vi "UHR-Fleezers Control (host) - 10.4.vi"() -> ()   [LabVIEW 2010] (continued)
              }
              frame #4 {
                n1609 = call "Write to pump.vi"("string"="start", "VISA resource name"=w7308) -> ()  [unwired: 1 out]
              }
            }
          }
        }
      }
      event "Inject Pump 2": Value Change {
        n1610 = event-data() -> ()  [unwired: 7 out]
        n1611 = local read "Pump write delay (ms)"() -> (w7312:dbl)
        n1612 = flat-sequence {
          tunnel: w7310 -> [w7325]
          tunnel: w7312 -> [w7321]
          tunnel: "Inject Pump 2" -> [_]
          tunnel: w7312 -> [w7327]
          tunnel: w7310 -> [w7328]
          frame #0 {
            n1613 = local read "All Pump Parameters"() -> (w7320:T6)
            n1614 = Multiply(x=60.0, y="Flush Center Ch Rate (ul/m)") -> (x*y=w7317:dbl)
            n1615 = Unbundle By Name(w7320) -> ("Pump 2"=w7326:T49)
            n1616 = call "Set pump parameters.vi"("Pump write delay (ms)"=w7321, "Volume (uL)"="Flush Center Ch Volume (uL)", "Rate (uL/h)"=w7317, "Units"=3.0, "Pump #"=2.0, "Pump Parameters In"=w7326, "VISA resource name"=w7325) -> ("Pump Parameters Out"=w7319:T49)  [unwired: 3 in]
            n1617 = Bundle By Name(cluster=w7320, "Pump 2"=w7319) -> (w7318:T6)
            n1618 = local write "All Pump Parameters"(w7318) -> ()
            n1619 = Add(x="Flush Center Ch Volume (uL)", y="Total Volume\nFlushed (uL)") -> (x+y=w7314:dbl)
            n1620 = local write "Total Volume\nFlushed (uL)"(w7314) -> ()
          }
          frame #1 {
            n1621 = Wait (ms)(milliseconds to wait=w7327) -> ()  [unwired: 1 out]
          }
          frame #2 {
            n1622 = call "Write to pump.vi"("string"="start", "VISA resource name"=w7328) -> ()  [unwired: 1 out]
          }
        }
        n1623 = local read "Chemyx Syringe Pump Serial Port"() -> (w7310:refnum<visa-resource-name>)
      }
      event "Sample Channel Flow": Value Change {
        n1624 = event-data() -> ()  [unwired: 7 out]
        n1625 = Select(t="run" ("string"), s="Sample Channel Flow", f="stop" ("string")) -> (s? t:f=w7330:string)
        n1626 = Concatenate Strings(w7330, "\r") -> (w7334:string)
        n1627 = VISA Write(VISA resource name=w7336, write buffer=w7334) -> ()  [unwired: 1 in, 3 out]
      }
      event "Flip Green Filter": Value Change {
        n1628 = event-data() -> ()  [unwired: 7 out]
        n1629 = Not(x="Flip Green Filter") -> (.not. x?=w7337:bool)
        n1630 = local write "Flip Green Filter"(w7337) -> ()
        n1631 = flat-sequence {
          tunnel: w7345 -> [w7350]
          tunnel: w7344 -> [w7349]
          tunnel: [w7347] -> w7342
          tunnel: [w7346] -> w7341
          tunnel: [w7390] -> w7340
          tunnel: w7342 -> [w7390]
          tunnel: [w7389] -> w7339
          tunnel: w7341 -> [w7389]
          tunnel: w7340 -> [w7394]
          tunnel: w7339 -> [w7393]
          tunnel: [w7392] -> w7343
          frame #0 {
            n1632 = xnode "Read/Write Control"("FPGA VI Reference In"=w7350, "error in"=w7349, "Green Filter Flipper"=TRUE) -> ("FPGA VI Reference Out"=w7347:T20, "error out"=w7346:errorcluster)
          }
          frame #1 {
            n1633 = Wait (ms)(milliseconds to wait=u32 100) -> ()  [unwired: 1 out]
          }
          frame #2 {
            n1634 = xnode "Read/Write Control"("FPGA VI Reference In"=w7394, "error in"=w7393, "Green Filter Flipper"=FALSE) -> ("error out"=w7392:errorcluster)  [unwired: 1 out]
          }
        }
      }
      event "Pump 1 contents", "Pump 3 contents": Value Change {
        n1635 = event-data() -> ()  [unwired: 7 out]
        n1636 = local read "Pump 1 contents"() -> (→"Pump 1 cont disp":string)
        n1637 = local read "Pump 3 contents"() -> (→"Pump 3 cont disp":string)
      }
      event "Reset Trap Pos. FB": Value Change {
        n1638 = event-data() -> ()  [unwired: 7 out]
        n1639 = xnode "Read/Write Control"("FPGA VI Reference In"=w7438, "error in"=w7437, "Trap Pos. FB Reset"="Reset Trap Pos. FB") -> ()  [unwired: 2 out]
      }
      event "Trap Pos. FB ON": Value Change {
        n1640 = event-data() -> ()  [unwired: 7 out]
        n1641 = xnode "Read/Write Control"("FPGA VI Reference In"=w7479, "error in"=w7478, "Force feedback"="Trap Pos. FB ON") -> ()  [unwired: 2 out]
      }
      event "Trap Pos. FB Range", "Trap Pos. FB Gains", "Trap Pos. FB Mult Factor", "Trap Pos. FB Offset Factor", "Trap Pos FB Negate Action", "Trap Pos FB Monitor\nT1 or T2": Value Change {
        n1642 = event-data() -> ()  [unwired: 7 out]
        n1643 = xnode "Read/Write Control"("FPGA VI Reference In"=w7526, "error in"=w7525, "Trap Pos. FB Range"="Trap Pos. FB Range", "Trap Pos. FB Gains"="Trap Pos. FB Gains", "Trap Pos. FB Mult Factor"="Trap Pos. FB Mult Factor", "Trap Pos. FB Offset Factor"="Trap Pos. FB Offset Factor", "Trap Pos FB Negate Action"="Trap Pos FB Negate Action", "Trap Pos FB Monitor T1 or T2"="Trap Pos FB Monitor\nT1 or T2", "AI1 X Scale"="Trap Pos. AI1 X Pre-scale") -> ()  [unwired: 2 out]
      }
      event "Trap Pos FB SP": Value Change {
        n1644 = event-data() -> ()  [unwired: 7 out]
        n1645 = xnode "Read/Write Control"("FPGA VI Reference In"=w7714, "error in"=w7713, "Trap Pos. FB SP"="Trap Pos FB SP") -> ()  [unwired: 2 out]
      }
      event "Set SP to Reading": Value Change {
        n1646 = event-data() -> ()  [unwired: 7 out]
        n1647 = local read "Trap Pos FB Monitor\nT1 or T2"() -> (w7767:bool)
        n1648 = local read "Trap X AI1 (DMA)"() -> (w7770:T14)
        n1649 = local read "Trap X (AI1)"() -> (w7773:T11)
        n1650 = Unbundle By Name(w7773) -> ("Trap 1"=w7772:fxp<+/-,16,1>, "Trap 2"=w7771:fxp<+/-,16,1>)
        n1651 = Unbundle By Name(w7770) -> ("Set 1"=w7769:fxp<+/-,16,1>, "Set 2"=w7768:fxp<+/-,16,1>)
        n1652 = Select(t=w7772, s=w7767, f=w7771) -> (s? t:f=w7766:fxp<+/-,16,1>)
        n1653 = Select(t=w7769, s=w7767, f=w7768) -> (s? t:f=w7765:fxp<+/-,16,1>)
        n1654 = Not(x="Set SP Using...") -> (.not. x?=w7760:bool)
        n1655 = Select(t=w7766, s=w7760, f=w7765) -> (s? t:f=w7761:fxp<+/-,16,1>)
        n1656 = xnode "Read/Write Control"("FPGA VI Reference In"=w7763, "error in"=w7762, "Trap Pos. FB SP"=w7761) -> ()  [unwired: 2 out]
        n1657 = local write "Trap Pos FB SP"(w7761) -> ()
      }
      event "Trap Pos. FB Out Scale 2^n": Value Change {
        n1658 = event-data() -> ()  [unwired: 7 out]
        n1659 = Scale By Power Of 2(n="Trap Pos. FB Out Scale 2^n", x=ext 1.0) -> (x*2^n=w7820:ext)
        n1660 = property on="Trap Pos. FB Mult Factor" class="DigNum (strict)"("Val(Sgnl)"=w7820) -> ()  [unwired: 2 in, 2 out]
      }
      event "Trap Pos FB Int Count": Value Change {
        n1661 = event-data() -> ()  [unwired: 7 out]
        n1662 = xnode "Read/Write Control"("FPGA VI Reference In"=w7825, "error in"=w7824, "Trap Pos FB Int Count"="Trap Pos FB Int Count") -> ()  [unwired: 2 out]
      }
    }
    "error out 2" <- w4314
    n1663 = node-c288() -> ()  [unwired: 2 out]
  }
  n1664 = timed-loop "Run Scripts, including: stage motion" {
    timing: w57 -> [_]
    timing-out: [_] -> w56
    tunnel: w42 -> [w7864]
    tunnel: w43 -> [w7863]
    stop <- w7865 stop-if-true
    n1665 = node-c288() -> ()  [unwired: 1 in, 1 out]
    n1666 = event shown="[6] \"Dump Beads\": Value Change" {
      selector: _ -> [_ _ _ _ _ _ _ _ _ _ _ _ _ _ _ _]
      dyn-events: _ -> [_ _ _ _ _ _ _ _ _ _ _ _ _ _ _ _]
      timeout: _ -> [_ _ _ _ _ _ _ _ _ _ _ _ _ _ _ _]
      tunnel: ["Set Position" "Move to Position" "Move Cap. 1 (DNA Right)" "Move Cap. 2 (ADig Left)" _ "Cal/Data Acq. Spot" "Dump Beads" "Dip for Protein" _ _ "Got ADig bead" "Got DNA bead" "Take Stepping Data" _ "Take Detection Laser\nImage" _] -> _
      tunnel: [_ _ _ _ _ _ _ _ _ _ _ _ _ _ _ w8280] -> w7865
      tunnel: w7864 -> [_ _ w7906 w7956 _ _ _ _ _ _ _ _ _ _ _ _]
      tunnel: w7863 -> [_ _ w7905 w7957 _ _ _ _ _ _ _ _ _ _ _ _]
      event "Set Position", "Set Position 2", "Set Position 3", "Set Position 4", "Set Position 5", "Set Position 1": Value Change {
        n1667 = event-data() -> ()  [unwired: 1 in, 5 out]
        n1668 = Build Array("Set Position 1", "Set Position 2", "Set Position 3", "Set Position 4", "Set Position 5") -> (w7884:bool[])
        n1669 = Boolean Array To Number(Boolean array=w7884) -> (number=w7883:u32)
        n1670 = Logarithm Base 2(1:w7883) -> (0:w7875:dbl)
        n1671 = call "CONEX_FUNCTIONAL_GLOBAL.vi"("Command"=T23."GET POS") -> ("Current Position"=w7868:dbl[])  [unwired: 8 in, 2 out]
        n1672 = Decrement(x="Position") -> (x-1=w7873:dbl)
        n1673 = Greater Or Equal?(x=w7875, y=0.0) -> (x >= y?=w7876:bool)
        n1674 = Select(t=w7875, s=w7876, f=w7873) -> (s? t:f=w7872:dbl)
        n1675 = Increment(x=w7872) -> (x+1=w7871:dbl)
        n1676 = Build Array (concatenate)(w7871, w7868) -> (w7870:dbl[])
        n1677 = Replace Array Subset(array="Saved Stage Positions", new element=w7870, index (row)=w7872) -> (w7885:dbl[][])  [unwired: 1 in]
        n1678 = local write "Saved Stage Positions"(w7885) -> ()
      }
      event "Move to Position": Value Change {
        n1679 = event-data() -> ()  [unwired: 1 in, 5 out]
        n1680 = flat-sequence {
          frame #0 {
            n1681 = local read "Position"() -> (w7900:dbl)
            n1682 = local read "Saved Stage Positions"() -> (w7898:dbl[][])
            n1683 = Decrement(x=w7900) -> (x-1=w7897:dbl)
            n1684 = Array Subset(array=w7898, index (row)=w7897, length (row)=1 ("length"), index (col)=1 ("index"), length (col)=3 ("length")) -> (w7894:dbl[][])
            n1685 = Reshape Array(w7894, 3 ("dimension size")) -> (w7890:dbl[])
            n1686 = local write "Stage Moving"(TRUE ("Stage Moving")) -> ()
            n1687 = call "CONEX_FUNCTIONAL_GLOBAL.vi"("Axis"=enum16{"X", "Y", "Z", "XY", "XZ", "YZ", "XYZ"}."XYZ", "Position"=w7890, "Command"=T23."ABS MOVE") -> ()  [unwired: 6 in, 3 out]
          }
          frame #1 {
            n1688 = call <vilib>:"Beep.vi"() -> ()  [unwired: 3 in, 9 out]
            n1689 = local write "Stage Moving"(FALSE ("Stage Moving")) -> ()
          }
        }
      }
      event "Move Cap. 1 (DNA Right)": Value Change {
        n1690 = event-data() -> ()  [unwired: 1 in, 5 out]
        n1691 = local write "Move Cap. 1 (DNA Right)"(FALSE ("Move Cap. 1 (DNA Right)")) -> ()
        n1692 = flat-sequence {
          tunnel: w7906 -> [w7916]
          tunnel: w7905 -> [w7915]
          tunnel: [w7914] -> w7904
          tunnel: [w7913] -> w7903
          tunnel: ["Cap 1 Samp Flow ON"] -> w7902
          tunnel: w7904 -> [w7936]
          tunnel: w7903 -> [w7935]
          tunnel: w7902 -> [w7934]
          frame #0 {
            n1693 = local read "Saved Stage Positions"() -> (w7923:dbl[][])
            n1694 = Array Subset(array=w7923, index (row)=0 ("index"), length (row)=1 ("length"), index (col)=1 ("index"), length (col)=3 ("length")) -> (w7920:dbl[][])
            n1695 = Reshape Array(w7920, 3 ("dimension size")) -> (w7910:dbl[])
            n1696 = case shown="True" "Cap 1 Samp Flow ON" {
              tunnel: w7915 -> [w7925 w7931]
              tunnel: w7916 -> [w7926 w7930]
              tunnel: [w7926 w7928] -> w7914
              tunnel: [w7925 w7927] -> w7913
              frame False {
              }
              frame True {
                # "run flow"
                n1697 = Concatenate Strings("run" ("string"), "\r") -> (w7932:string)
                n1698 = VISA Write(VISA resource name=w7930, write buffer=w7932, error in (no error)=w7931) -> (VISA resource name out=w7928:refnum<visa-resource-name>, error out=w7927:errorcluster)  [unwired: 1 out]
              }
            }
            n1699 = call "CONEX_FUNCTIONAL_GLOBAL.vi"("Axis"=enum16{"X", "Y", "Z", "XY", "XZ", "YZ", "XYZ"}."XYZ", "Position"=w7910, "Command"=T23."ABS MOVE") -> ()  [unwired: 6 in, 3 out]
            n1700 = local write "Stage Moving"(TRUE ("Stage Moving")) -> ()
          }
          frame #1 {
            n1701 = local write "Stage Moving"(FALSE ("Stage Moving")) -> ()
            n1702 = case shown="True" w7934 {
              tunnel: w7935 -> [w7941 w7947]
              tunnel: w7936 -> [w7942 w7946]
              tunnel: [w7942 w7944] -> _
              tunnel: [w7941 w7943] -> _
              frame False {
              }
              frame True {
                n1703 = Concatenate Strings("stop" ("string"), "\r") -> (w7948:string)
                n1704 = VISA Write(VISA resource name=w7946, write buffer=w7948, error in (no error)=w7947) -> (VISA resource name out=w7944:refnum<visa-resource-name>, error out=w7943:errorcluster)  [unwired: 1 out]
              }
            }
            n1705 = case shown="True" TRUE {
              tunnel: "Cap 1 T ON" -> [w7951 w7952]
              frame False {
                n1706 = property on="Trap 1 (ON/OFF)" class="Bool (strict)"("Val(Sgnl)"=w7951) -> ()  [unwired: 2 in, 2 out]
              }
              frame True {
                n1707 = property on="Trap 2 (ON/OFF)" class="Bool (strict)"("Val(Sgnl)"=w7952) -> ()  [unwired: 2 in, 2 out]
              }
            }
            n1708 = call <vilib>:"Beep.vi"() -> ()  [unwired: 3 in, 9 out]
            n1709 = case shown="True" "Cap 1 Flow ON" {
              frame False {
              }
              frame True {
                n1710 = property on="Inject Pump 1" class="Bool (strict)"("Val(Sgnl)"=TRUE ("Value (Signaling)")) -> ()  [unwired: 2 in, 2 out]
              }
            }
          }
        }
      }
      event "Move Cap. 2 (ADig Left)": Value Change {
        n1711 = event-data() -> ()  [unwired: 1 in, 5 out]
        n1712 = local write "Move Cap. 2 (ADig Left)"(FALSE ("Move Cap. 2 (ADig Left)")) -> ()
        n1713 = flat-sequence {
          tunnel: w7957 -> [w7967]
          tunnel: w7956 -> [w7966]
          tunnel: [w7965] -> w7955
          tunnel: [w7964] -> w7954
          tunnel: ["Cap 2 Samp Flow ON"] -> w7953
          tunnel: w7955 -> [w7987]
          tunnel: w7954 -> [w7986]
          tunnel: w7953 -> [w7985]
          frame #0 {
            n1714 = local read "Saved Stage Positions"() -> (w7974:dbl[][])
            n1715 = case shown="True" "Cap 2 Samp Flow ON" {
              tunnel: w7967 -> [w7976 w7982]
              tunnel: w7966 -> [w7977 w7981]
              tunnel: [w7977 w7979] -> w7965
              tunnel: [w7976 w7978] -> w7964
              frame False {
              }
              frame True {
                # "run flow"
                n1716 = Concatenate Strings("run" ("string"), "\r") -> (w7983:string)
                n1717 = VISA Write(VISA resource name=w7981, write buffer=w7983, error in (no error)=w7982) -> (VISA resource name out=w7979:refnum<visa-resource-name>, error out=w7978:errorcluster)  [unwired: 1 out]
              }
            }
            n1718 = Array Subset(array=w7974, index (row)=1 ("index"), length (row)=1 ("length"), index (col)=1 ("index"), length (col)=3 ("length")) -> (w7971:dbl[][])
            n1719 = Reshape Array(w7971, 3 ("dimension size")) -> (w7961:dbl[])
            n1720 = local write "Stage Moving"(TRUE ("Stage Moving")) -> ()
            n1721 = call "CONEX_FUNCTIONAL_GLOBAL.vi"("Axis"=enum16{"X", "Y", "Z", "XY", "XZ", "YZ", "XYZ"}."XYZ", "Position"=w7961, "Command"=T23."ABS MOVE") -> ()  [unwired: 6 in, 3 out]
          }
          frame #1 {
            n1722 = local write "Stage Moving"(FALSE ("Stage Moving")) -> ()
            n1723 = case shown="True" TRUE {
              tunnel: "Cap 2 T ON" -> [w7998 w7999]
              frame False {
                n1724 = property on="Trap 2 (ON/OFF)" class="Bool (strict)"("Val(Sgnl)"=w7998) -> ()  [unwired: 2 in, 2 out]
              }
              frame True {
                n1725 = property on="Trap 1 (ON/OFF)" class="Bool (strict)"("Val(Sgnl)"=w7999) -> ()  [unwired: 2 in, 2 out]
              }
            }
            n1726 = call <vilib>:"Beep.vi"() -> ()  [unwired: 3 in, 9 out]
            n1727 = case shown="True" w7985 {
              tunnel: w7987 -> [_ w7993]
              tunnel: w7986 -> [_ w7992]
              frame False {
              }
              frame True {
                n1728 = Concatenate Strings("stop" ("string"), "\r") -> (w7995:string)
                n1729 = VISA Write(VISA resource name=w7993, write buffer=w7995, error in (no error)=w7992) -> ()  [unwired: 3 out]
              }
            }
            n1730 = case shown="True" "Cap 2 Flow ON" {
              frame False {
              }
              frame True {
                n1731 = property on="Inject Pump 3" class="Bool (strict)"("Val(Sgnl)"=TRUE ("Value (Signaling)")) -> ()  [unwired: 2 in, 2 out]
              }
            }
          }
        }
      }
      event "+z", "-z": Value Change {
        n1732 = event-data() -> ()  [unwired: 1 in, 5 out]
        n1733 = flat-sequence {
          frame #0 {
            w8001 = 0.0 ("element")
            n1734 = Divide(x="z nudge increment (um)", y=1000.0) -> (x/y=w8014:dbl)
            n1735 = Boolean To (0,1)(Boolean="+z") -> (0, 1=w8007:i16)
            n1736 = Boolean To (0,1)(Boolean="-z") -> (0, 1=w8008:i16)
            n1737 = Multiply(x=w8007, y=w8014) -> (x*y=w8011:dbl)
            n1738 = Multiply(x=w8008, y=w8014) -> (x*y=w8009:dbl)
            n1739 = Negate(x=w8009) -> (-x=w8010:dbl)
            n1740 = Add(x=w8011, y=w8010) -> (x+y=w8002:dbl)
            n1741 = Build Array(w8001, w8001, w8002) -> (w8000:dbl[])
            n1742 = call "CONEX_FUNCTIONAL_GLOBAL.vi"("Axis"=enum16{"X", "Y", "Z", "XY", "XZ", "YZ", "XYZ"}."Z", "Position"=w8000, "Command"=T23."REL MOVE") -> ()  [unwired: 6 in, 3 out]
            n1743 = local write "Stage Moving"(TRUE ("Stage Moving")) -> ()
          }
          frame #1 {
            n1744 = local write "Stage Moving"(FALSE ("Stage Moving")) -> ()
            n1745 = call <vilib>:"Beep.vi"() -> ()  [unwired: 3 in, 9 out]
          }
        }
      }
      event "Cal/Data Acq. Spot": Value Change {
        n1746 = event-data() -> ()  [unwired: 1 in, 5 out]
        n1747 = flat-sequence {
          tunnel: ["Cal @ (MHz)"] -> w8017
          tunnel: w8017 -> [w8039]
          tunnel: w8017 -> [w8060]
          frame #0 {
            n1748 = local read "Saved Stage Positions"() -> (w8025:dbl[][])
            n1749 = Array Subset(array=w8025, index (row)=2 ("index"), length (row)=1 ("length"), index (col)=1 ("index"), length (col)=3 ("length")) -> (w8028:dbl[][])
            n1750 = Reshape Array(w8028, 3 ("dimension size")) -> (w8021:dbl[])
            n1751 = local write "Stage Moving"(TRUE ("Stage Moving")) -> ()
            n1752 = call "CONEX_FUNCTIONAL_GLOBAL.vi"("Axis"=enum16{"X", "Y", "Z", "XY", "XZ", "YZ", "XYZ"}."XYZ", "Position"=w8021, "Command"=T23."ABS MOVE") -> ()  [unwired: 6 in, 3 out]
          }
          frame #1 {
            n1753 = property on="Trap Delta (MHz)" class="DigNum (strict)"("Val(Sgnl)"="Cal @ (MHz)") -> ()  [unwired: 2 in, 2 out]
            n1754 = local write "Stage Moving"(FALSE ("Stage Moving")) -> ()
            n1755 = call <vilib>:"Beep.vi"() -> ()  [unwired: 3 in, 9 out]
          }
          frame #2 {
            n1756 = Wait (ms)(milliseconds to wait=u32 100) -> ()  [unwired: 1 out]
          }
          frame #3 {
            n1757 = property on="Save Calibration" class="Bool (strict)"("Val(Sgnl)"=TRUE ("Value (Signaling)")) -> ()  [unwired: 2 in, 2 out]
          }
          frame #4 {
            n1758 = Wait (ms)(milliseconds to wait=u32 4000) -> ()  [unwired: 1 out]
          }
          frame #5 {
            n1759 = while {
              stop <- w8036 stop-if-true
              n1760 = local read "Saving..."() -> (w8037:bool)
              n1761 = Wait (ms)(milliseconds to wait=u32 100) -> ()  [unwired: 1 out]
              n1762 = Not(x=w8037) -> (.not. x?=w8036:bool)
            }
          }
          frame #6 {
            n1763 = case shown="True" "W/ Offset 1" {
              tunnel: w8039 -> [_ w8041]
              frame False {
              }
              frame True {
                n1764 = stacked-sequence {
                  tunnel: w8041 -> [_ _ _ _ _ _ _ w8058]
                  frame #0 {
                    n1765 = property on="Trap Delta (MHz)" class="DigNum (strict)"("Val(Sgnl)"="Offset 1 Start (MHz)") -> ()  [unwired: 2 in, 2 out]
                    n1766 = Replace Array Subset(array=u32[] [0] ("Index Values"), new element="Offset 1 Set", index=0) -> (w8042:u32[])
                    n1767 = property on="Saved AOD Raster Scan Parameter Sets" class="Arr (strict)"("Index Values"=w8042) -> ()  [unwired: 2 in, 2 out]
                  }
                  frame #1 {
                    n1768 = Wait (ms)(milliseconds to wait=u32 200) -> ()  [unwired: 1 out]
                  }
                  frame #2 {
                    n1769 = property on="Load parameters" class="Bool (strict)"("Val(Sgnl)"=TRUE ("Value (Signaling)")) -> ()  [unwired: 2 in, 2 out]
                  }
                  frame #3 {
                    n1770 = Wait (ms)(milliseconds to wait=u32 200) -> ()  [unwired: 1 out]
                  }
                  frame #4 {
                    n1771 = property on="Trap Raster Scan" class="Bool (strict)"("Val(Sgnl)"=TRUE ("Value (Signaling)")) -> ()  [unwired: 2 in, 2 out]
                  }
                  frame #5 {
                    n1772 = Wait (ms)(milliseconds to wait=u32 2000) -> ()  [unwired: 1 out]
                  }
                  frame #6 {
                    n1773 = while {
                      stop <- w8055 stop-if-true
                      n1774 = local read "Raster Scanning..."() -> (w8057:bool)
                      n1775 = local read "Saving..."() -> (w8053:bool)
                      n1776 = Wait (ms)(milliseconds to wait=u32 100) -> ()  [unwired: 1 out]
                      n1777 = Not(x=w8053) -> (.not. x?=w8052:bool)
                      n1778 = Not(x=w8057) -> (.not. x?=w8054:bool)
                      n1779 = And(x=w8054, y=w8052) -> (x .and. y?=w8055:bool)
                    }
                  }
                  frame #7 {
                    n1780 = property on="Trap Delta (MHz)" class="DigNum (strict)"("Val(Sgnl)"=w8058) -> ()  [unwired: 2 in, 2 out]
                  }
                }
              }
            }
          }
          frame #7 {
            n1781 = local read "Save ave N"() -> (w8059:dbl)
            n1782 = case shown="True" "W/ Offset 2" {
              tunnel: w8060 -> [_ w8066]
              tunnel: w8059 -> [_ w8065]
              frame False {
                n1783 = Multiply(x="Cal read wait (s)", y=u32 1000 ("milliseconds to wait")) -> (x*y=w8063:u32)
                n1784 = Wait (ms)(milliseconds to wait=w8063) -> ()  [unwired: 1 out]
              }
              frame True {
                n1785 = stacked-sequence {
                  tunnel: w8066 -> [_ _ _ _ _ _ _ _ _ w8087 _ _]
                  tunnel: w8065 -> [_ _ _ _ _ _ _ _ _ w8085 _ _]
                  frame #0 {
                    n1786 = property on="Save ave N" class="DigNum (strict)"("Val(Sgnl)"=1.0 ("Value (Signaling)")) -> ()  [unwired: 2 in, 2 out]
                  }
                  frame #1 {
                    n1787 = Wait (ms)(milliseconds to wait=u32 500) -> ()  [unwired: 1 out]
                  }
                  frame #2 {
                    n1788 = property on="Trap Delta (MHz)" class="DigNum (strict)"("Val(Sgnl)"="Offset 2 Start (MHz)") -> ()  [unwired: 2 in, 2 out]
                    n1789 = Replace Array Subset(array=u32[] [0] ("Index Values"), new element="Offset 2 Set", index=0) -> (w8071:u32[])
                    n1790 = property on="Saved AOD Raster Scan Parameter Sets" class="Arr (strict)"("Index Values"=w8071) -> ()  [unwired: 2 in, 2 out]
                  }
                  frame #3 {
                    n1791 = Wait (ms)(milliseconds to wait=u32 500) -> ()  [unwired: 1 out]
                  }
                  frame #4 {
                    n1792 = property on="Load parameters" class="Bool (strict)"("Val(Sgnl)"=TRUE ("Value (Signaling)")) -> ()  [unwired: 2 in, 2 out]
                  }
                  frame #5 {
                    n1793 = Wait (ms)(milliseconds to wait=u32 500) -> ()  [unwired: 1 out]
                  }
                  frame #6 {
                    n1794 = property on="Trap Raster Scan" class="Bool (strict)"("Val(Sgnl)"=TRUE ("Value (Signaling)")) -> ()  [unwired: 2 in, 2 out]
                  }
                  frame #7 {
                    n1795 = Wait (ms)(milliseconds to wait=u32 2000) -> ()  [unwired: 1 out]
                  }
                  frame #8 {
                    n1796 = while {
                      stop <- w8080 stop-if-true
                      n1797 = local read "Raster Scanning..."() -> (w8083:bool)
                      n1798 = local read "Saving..."() -> (w8081:bool)
                      n1799 = Wait (ms)(milliseconds to wait=u32 100) -> ()  [unwired: 1 out]
                      n1800 = Not(x=w8081) -> (.not. x?=w8079:bool)
                      n1801 = Not(x=w8083) -> (.not. x?=w8082:bool)
                      n1802 = And(x=w8082, y=w8079) -> (x .and. y?=w8080:bool)
                    }
                  }
                  frame #9 {
                    n1803 = property on="Trap Delta (MHz)" class="DigNum (strict)"("Val(Sgnl)"=w8087) -> ()  [unwired: 2 in, 2 out]
                    n1804 = property on="Saved AOD Raster Scan Parameter Sets" class="Arr (strict)"("Index Values"=u32[] [0]) -> ()  [unwired: 2 in, 2 out]
                    n1805 = property on="Save ave N" class="DigNum (strict)"("Val(Sgnl)"=w8085) -> ()  [unwired: 2 in, 2 out]
                  }
                  frame #10 {
                    n1806 = Wait (ms)(milliseconds to wait=u32 500) -> ()  [unwired: 1 out]
                  }
                  frame #11 {
                    n1807 = property on="Load parameters" class="Bool (strict)"("Val(Sgnl)"=TRUE ("Value (Signaling)")) -> ()  [unwired: 2 in, 2 out]
                  }
                }
              }
            }
          }
          frame #8 {
            n1808 = property on="Read Cal" class="Bool (strict)"("Val(Sgnl)"=TRUE ("Value (Signaling)")) -> ()  [unwired: 2 in, 2 out]
          }
          frame #9 {
            n1809 = Wait (ms)(milliseconds to wait=u32 500) -> ()  [unwired: 1 out]
          }
          frame #10 {
            n1810 = property on="Fish for Tether" class="Bool (strict)"("Val(Sgnl)"=TRUE ("Value (Signaling)")) -> ()  [unwired: 2 in, 2 out]
          }
        }
        n1811 = local write "Cal/Data Acq. Spot"(FALSE ("Cal/Data Acq. Spot")) -> ()
      }
      event "Dump Beads": Value Change {
        # "SCRIPT TO REMOVE BOTH BEADS FROM THE TRAPS. TURNS ON LIGHT WHICH INDICATES THAT STAGE IS MOVING. THEN STOPS SAVING DATA. \nSETS Sample Channel Flow TO TRUE. STOPS INTERLACING GREEN FLUORESCENCE. TURNS OFF Tether INDICATOR BECAUSE WE ARE THROWING IT\nAWAY. SHUTS OFF TRAP POSITION FEEDBACK."
        n1812 = event-data() -> ()  [unwired: 1 in, 5 out]
        n1813 = flat-sequence {
          frame #0 {
            w8094 = FALSE ("Fl. Triggered...")
            w8095 = TRUE ("Stage Moving")
            n1814 = local read "Saving..."() -> (w8096:bool)
            n1815 = local write "Fl. Triggered..."(w8094) -> ()
            n1816 = local write "Stage Moving"(w8095) -> ()
            n1817 = local write "Tether"(w8094) -> ()
            n1818 = property on="Green Laser ON/Interlacing" class="Bool (strict)"("Val(Sgnl)"=w8094) -> ()  [unwired: 2 in, 2 out]
            n1819 = property on="Trap Pos. FB ON" class="Bool (strict)"("Val(Sgnl)"=w8094) -> ()  [unwired: 2 in, 2 out]
            n1820 = property on="Sample Channel Flow" class="Bool (strict)"("Val(Sgnl)"=w8095) -> ()  [unwired: 2 in, 2 out]
            n1821 = local write "Stop Saving"(w8096) -> ()
          }
          frame #1 {
            # "MOVES TO THE DUMP BEADS POSITION"
            n1822 = local read "Saved Stage Positions"() -> (w8100:dbl[][])
            n1823 = Array Subset(array=w8100, index (row)=3 ("index"), length (row)=1 ("length"), index (col)=1 ("index"), length (col)=3 ("length")) -> (w8103:dbl[][])
            n1824 = Reshape Array(w8103, 3 ("dimension size")) -> (w8098:dbl[])
            n1825 = call "CONEX_FUNCTIONAL_GLOBAL.vi"("Axis"=enum16{"X", "Y", "Z", "XY", "XZ", "YZ", "XYZ"}."XYZ", "Position"=w8098, "Command"=T23."ABS MOVE") -> ()  [unwired: 6 in, 3 out]
          }
          frame #2 {
            w8107 = FALSE ("Value (Signaling)")
            # "TURNS TRAPS OFF SO THAT\nBEADS REMAIN AT DUMP \nBEADS POSITION"
            n1826 = property on="Trap 1 (ON/OFF)" class="Bool (strict)"("Val(Sgnl)"=w8107) -> ()  [unwired: 2 in, 2 out]
            n1827 = property on="Trap 2 (ON/OFF)" class="Bool (strict)"("Val(Sgnl)"=w8107) -> ()  [unwired: 2 in, 2 out]
            n1828 = call <vilib>:"Beep.vi"() -> ()  [unwired: 3 in, 9 out]
          }
          frame #3 {
            # "MOVES STAGE BACK TO THE\nANTIDIG CAPILARY BY CALLING\nTHE Move Cap. 2 SCRIPT"
            n1829 = property on="Move Cap. 2 (ADig Left)" class="Bool (strict)"("Val(Sgnl)"=TRUE ("Value (Signaling)")) -> ()  [unwired: 2 in, 2 out]
          }
        }
      }
      event "Dip for Protein": Value Change {
        n1830 = event-data() -> ()  [unwired: 1 in, 5 out]
        n1831 = flat-sequence {
          frame #0 {
            n1832 = case shown="True" "Move Trap Before?" {
              frame False {
              }
              frame True {
                n1833 = property on="Trap Delta (MHz)" class="DigNum (strict)"("Val(Sgnl)"="Dip Trap Delta 1 (MHz)") -> ()  [unwired: 2 in, 2 out]
              }
            }
          }
          frame #1 {
            n1834 = local read "Saved Stage Positions"() -> (w8115:dbl[][])
            n1835 = Array Subset(array=w8115, index (row)=4 ("index"), length (row)=1 ("length"), index (col)=1 ("index"), length (col)=3 ("length")) -> (w8118:dbl[][])
            n1836 = Reshape Array(w8118, 3 ("dimension size")) -> (w8113:dbl[])
            n1837 = call "CONEX_FUNCTIONAL_GLOBAL.vi"("Axis"=enum16{"X", "Y", "Z", "XY", "XZ", "YZ", "XYZ"}."XYZ", "Position"=w8113, "Command"=T23."ABS MOVE") -> ()  [unwired: 6 in, 3 out]
          }
          frame #2 {
            n1838 = Multiply(x="Duration (s)", y=1000.0) -> (x*y=w8122:dbl)
            n1839 = Wait (ms)(milliseconds to wait=w8122) -> ()  [unwired: 1 out]
          }
          frame #3 {
            n1840 = local read "Saved Stage Positions"() -> (w8128:dbl[][])
            n1841 = Array Subset(array=w8128, index (row)=2 ("index"), length (row)=1 ("length"), index (col)=1 ("index"), length (col)=3 ("length")) -> (w8131:dbl[][])
            n1842 = Reshape Array(w8131, 3 ("dimension size")) -> (w8126:dbl[])
            n1843 = call "CONEX_FUNCTIONAL_GLOBAL.vi"("Axis"=enum16{"X", "Y", "Z", "XY", "XZ", "YZ", "XYZ"}."XYZ", "Position"=w8126, "Command"=T23."ABS MOVE") -> ()  [unwired: 6 in, 3 out]
          }
          frame #4 {
            n1844 = case shown="True" "Move Trap After?" {
              frame False {
              }
              frame True {
                n1845 = property on="Trap Delta (MHz)" class="DigNum (strict)"("Val(Sgnl)"="Dip Trap Delta 2 (MHz)") -> ()  [unwired: 2 in, 2 out]
              }
            }
          }
          frame #5 {
            n1846 = case shown="True" "Green ON After?" {
              frame False {
              }
              frame True {
                n1847 = property on="Green Laser ON/Interlacing" class="Bool (strict)"("Val(Sgnl)"=TRUE ("Value (Signaling)")) -> ()  [unwired: 2 in, 2 out]
              }
            }
          }
          frame #6 {
            n1848 = Wait (ms)(milliseconds to wait=u32 500) -> ()  [unwired: 1 out]
          }
          frame #7 {
            n1849 = case shown="True" "Save Data After?" {
              frame False {
              }
              frame True {
                n1850 = property on="Start Saving" class="Bool (strict)"("Val(Sgnl)"=TRUE ("Value (Signaling)")) -> ()  [unwired: 2 in, 2 out]
              }
            }
          }
        }
      }
      event "Profile": Value Change {
        n1851 = event-data() -> ()  [unwired: 1 in, 5 out]
        n1852 = flat-sequence {
          tunnel: [w8144] -> w8143
          tunnel: w8143 -> [w8148]
          tunnel: [w8147] -> w8142
          tunnel: w8142 -> [w8154]
          frame #0 {
            w8145 = 0.0 ("element")
            n1853 = Build Array(w8145, "Y change (mm)", w8145) -> (w8144:dbl[])
          }
          frame #1 {
            # "move to new position and start saving"
            n1854 = local write "Stage Moving"(TRUE ("Stage Moving")) -> ()
            n1855 = local write "Start Saving"(TRUE ("Start Saving")) -> ()
            n1856 = call "CONEX_FUNCTIONAL_GLOBAL.vi"("Axis"=enum16{"X", "Y", "Z", "XY", "XZ", "YZ", "XYZ"}."Y", "Position"=w8148, "Command"=T23."REL MOVE") -> ()  [unwired: 6 in, 3 out]
            n1857 = Negate(x=w8148) -> (-x=w8147:dbl[])
          }
          frame #2 {
            # "go back to start"
            n1858 = call "CONEX_FUNCTIONAL_GLOBAL.vi"("Axis"=enum16{"X", "Y", "Z", "XY", "XZ", "YZ", "XYZ"}."Y", "Position"=w8154, "Command"=T23."REL MOVE") -> ()  [unwired: 6 in, 3 out]
          }
          frame #3 {
            # "stop saving"
            n1859 = local write "Stop Saving"(TRUE ("Stop Saving")) -> ()
            n1860 = local write "Stage Moving"(FALSE ("Stage Moving")) -> ()
          }
        }
      }
      event "Move to Position 1", "Move to Position 2", "Move to Position 3", "Move to Position 4", "Move to Position 5", "Lower Ch. Cap.": Value Change {
        n1861 = event-data() -> ()  [unwired: 1 in, 5 out]
        n1862 = Or(x="Move to Position 5", y="Lower Ch. Cap.") -> (x .or. y?=w8159:bool)
        n1863 = Build Array("Move to Position 1", "Move to Position 2", "Move to Position 3", "Move to Position 4", w8159) -> (w8162:bool[])
        n1864 = Boolean Array To Number(Boolean array=w8162) -> (number=w8161:u32)
        n1865 = Logarithm Base 2(1:w8161) -> (0:w8160:dbl)
        n1866 = flat-sequence {
          tunnel: w8160 -> [w8172]
          frame #0 {
            n1867 = local read "Saved Stage Positions"() -> (w8177:dbl[][])
            n1868 = Array Subset(array=w8177, index (row)=w8172, length (row)=1 ("length"), index (col)=1 ("index"), length (col)=3 ("length")) -> (w8174:dbl[][])
            n1869 = Reshape Array(w8174, 3 ("dimension size")) -> (w8169:dbl[])
            n1870 = local write "Stage Moving"(TRUE ("Stage Moving")) -> ()
            n1871 = call "CONEX_FUNCTIONAL_GLOBAL.vi"("Axis"=enum16{"X", "Y", "Z", "XY", "XZ", "YZ", "XYZ"}."XYZ", "Position"=w8169, "Command"=T23."ABS MOVE") -> ()  [unwired: 6 in, 3 out]
          }
          frame #1 {
            n1872 = local write "Stage Moving"(FALSE ("Stage Moving")) -> ()
            n1873 = call <vilib>:"Beep.vi"() -> ()  [unwired: 3 in, 9 out]
          }
        }
      }
      event "Got ADig bead": Value Change {
        n1874 = event-data() -> ()  [unwired: 1 in, 5 out]
        n1875 = property on="Move Cap. 1 (DNA Right)" class="Bool (strict)"("Val(Sgnl)"=TRUE ("Value (Signaling)")) -> ()  [unwired: 2 in, 2 out]
        n1876 = property on="Inject Pump 3" class="Bool (strict)"("Val(Sgnl)"=FALSE ("Value (Signaling)")) -> ()  [unwired: 2 in, 2 out]
      }
      event "Got DNA bead": Value Change {
        n1877 = event-data() -> ()  [unwired: 1 in, 5 out]
        n1878 = property on="Cal/Data Acq. Spot" class="Bool (strict)"("Val(Sgnl)"=TRUE ("Value (Signaling)")) -> ()  [unwired: 2 in, 2 out]
        n1879 = property on="Inject Pump 1" class="Bool (strict)"("Val(Sgnl)"=FALSE ("Value (Signaling)")) -> ()  [unwired: 2 in, 2 out]
      }
      event "Take Stepping Data": Value Change {
        n1880 = event-data() -> ()  [unwired: 1 in, 5 out]
        n1881 = local read "Save ave N"() -> (w8194:dbl)
        n1882 = flat-sequence {
          tunnel: w8194 -> [w8196]
          tunnel: [w8196] -> w8189
          tunnel: [w8198] -> w8190
          tunnel: w8189 -> [w8198]
          tunnel: [w8200] -> w8191
          tunnel: w8190 -> [w8200]
          tunnel: [w8203] -> w8192
          tunnel: w8191 -> [w8203]
          tunnel: [w8205] -> w8193
          tunnel: w8192 -> [w8205]
          tunnel: [w8207] -> w8187
          tunnel: w8193 -> [w8207]
          tunnel: w8187 -> [w8210]
          tunnel: [w8210] -> w8186
          tunnel: w8186 -> [w8211]
          tunnel: [w8211] -> w8188
          tunnel: w8188 -> [w8217]
          frame #0 {
            n1883 = property on="Save ave N" class="DigNum (strict)"("Val(Sgnl)"="Save ave factor") -> ()  [unwired: 2 in, 2 out]
          }
          frame #1 {
            n1884 = Wait (ms)(milliseconds to wait=u32 100) -> ()  [unwired: 1 out]
          }
          frame #2 {
            n1885 = local read "Offset 2 Start (MHz)"() -> (w8202:dbl)
            n1886 = property on="Saved AOD Raster Scan Parameter Sets" class="Arr (strict)"("Index Values"=u32[] [2]) -> ()  [unwired: 2 in, 2 out]
            n1887 = property on="Trap Delta (MHz)" class="DigNum (strict)"("Val(Sgnl)"=w8202) -> ()  [unwired: 2 in, 2 out]
          }
          frame #3 {
            n1888 = property on="Load parameters" class="Bool (strict)"("Val(Sgnl)"=TRUE ("Value (Signaling)")) -> ()  [unwired: 2 in, 2 out]
          }
          frame #4 {
            n1889 = Wait (ms)(milliseconds to wait=u32 100) -> ()  [unwired: 1 out]
          }
          frame #5 {
            n1890 = property on="Trap Raster Scan" class="Bool (strict)"("Val(Sgnl)"=TRUE ("Value (Signaling)")) -> ()  [unwired: 2 in, 2 out]
          }
          frame #6 {
            n1891 = Wait (ms)(milliseconds to wait=u32 1000) -> ()  [unwired: 1 out]
          }
          frame #7 {
            n1892 = while {
              stop <- w8214 stop-if-true
              n1893 = local read "Raster Scanning..."() -> (w8216:bool)
              n1894 = local read "Saving..."() -> (w8215:bool)
              n1895 = Not(x=w8215) -> (.not. x?=w8212:bool)
              n1896 = Not(x=w8216) -> (.not. x?=w8213:bool)
              n1897 = And(x=w8213, y=w8212) -> (x .and. y?=w8214:bool)
            }
          }
          frame #8 {
            n1898 = property on="Save ave N" class="DigNum (strict)"("Val(Sgnl)"=w8217) -> ()  [unwired: 2 in, 2 out]
          }
        }
      }
      event "Step Size (nm)": Value Change {
        n1899 = event-data() -> ()  [unwired: 1 in, 5 out]
        n1900 = flat-sequence {
          frame #0 {
            n1901 = property on="Saved AOD Raster Scan Parameter Sets" class="Arr (strict)"("Index Values"=u32[] [1]) -> ()  [unwired: 2 in, 2 out]
          }
          frame #1 {
            n1902 = Multiply(x="N Steps", y="Step Size (nm)") -> (x*y=w8219:dbl)
            n1903 = property on="Scan Speed AOD (nm/s) 2" class="DigNum (strict)"("Value"="Step Size (nm)") -> ()  [unwired: 2 in, 2 out]
            n1904 = property on="Step Size AOD (nm) 2" class="DigNum (strict)"("Value"="Step Size (nm)") -> ()  [unwired: 2 in, 2 out]
            n1905 = property on="Scan Range AOD (nm) 2" class="DigNum (strict)"("Value"=w8219) -> ()  [unwired: 2 in, 2 out]
          }
        }
      }
      event "Take Detection Laser\nImage": Value Change {
        n1906 = event-data() -> ()  [unwired: 1 in, 5 out]
        n1907 = flat-sequence {
          tunnel: [w8247] -> w8237
          tunnel: [w8246] -> w8230
          tunnel: [w8245] -> w8222
          tunnel: [w8250] -> w8238
          tunnel: w8237 -> [w8250]
          tunnel: [w8249] -> w8231
          tunnel: w8230 -> [w8249]
          tunnel: [w8248] -> w8223
          tunnel: w8222 -> [w8248]
          tunnel: [w8254] -> w8239
          tunnel: w8238 -> [w8254]
          tunnel: [w8253] -> w8232
          tunnel: w8231 -> [w8253]
          tunnel: [w8252] -> w8224
          tunnel: w8223 -> [w8252]
          tunnel: [w8260] -> w8240
          tunnel: w8239 -> [w8260]
          tunnel: [w8259] -> w8233
          tunnel: w8232 -> [w8259]
          tunnel: [w8258] -> w8225
          tunnel: w8224 -> [w8258]
          tunnel: [w8264] -> w8241
          tunnel: w8240 -> [w8264]
          tunnel: [w8263] -> w8234
          tunnel: w8233 -> [w8263]
          tunnel: [w8262] -> w8226
          tunnel: w8225 -> [w8262]
          tunnel: [w8268] -> w8242
          tunnel: w8241 -> [w8268]
          tunnel: [w8267] -> w8235
          tunnel: w8234 -> [w8267]
          tunnel: [w8266] -> w8227
          tunnel: w8226 -> [w8266]
          tunnel: [w8272] -> w8243
          tunnel: w8242 -> [w8272]
          tunnel: [w8271] -> w8236
          tunnel: w8235 -> [w8271]
          tunnel: [w8270] -> w8228
          tunnel: w8227 -> [w8270]
          tunnel: w8243 -> [w8278]
          tunnel: w8236 -> [w8277]
          tunnel: [w8275] -> w8229
          tunnel: w8228 -> [w8275]
          tunnel: w8229 -> [w8279]
          frame #0 {
            n1908 = local read "Green Laser ON/Interlacing"() -> (w8247:bool)
            n1909 = local read "Green laser mode"() -> (w8246:enum32{"Laser ON", "Laser OFF", "Interlace"})
            n1910 = local read "Green FB On/Off"() -> (w8245:bool)
          }
          frame #1 {
            n1911 = property on="Green FB On/Off" class="Bool (strict)"("Val(Sgnl)"=FALSE ("Value (Signaling)")) -> ()  [unwired: 2 in, 2 out]
          }
          frame #2 {
            n1912 = property on="Green Laser ON/Interlacing" class="Bool (strict)"("Val(Sgnl)"=TRUE ("Value (Signaling)")) -> ()  [unwired: 2 in, 2 out]
            n1913 = property on="Flip Green Filter" class="Bool (strict)"("Val(Sgnl)"=TRUE ("Value (Signaling)")) -> ()  [unwired: 2 in, 2 out]
            n1914 = property on="Green laser mode" class="RadioBtnsControl (strict)"("Val(Sgnl)"=enum32{"Laser ON", "Laser OFF", "Interlace"}."Laser ON" ("Value (Signaling)")) -> ()  [unwired: 2 in, 2 out]
          }
          frame #3 {
            n1915 = Wait (ms)(milliseconds to wait=u32 500) -> ()  [unwired: 1 out]
          }
          frame #4 {
            n1916 = property on="Confocal Image" class="Bool (strict)"("Val(Sgnl)"=TRUE ("Value (Signaling)")) -> ()  [unwired: 2 in, 2 out]
          }
          frame #5 {
            n1917 = Wait (ms)(milliseconds to wait=u32 2000) -> ()  [unwired: 1 out]
          }
          frame #6 {
            n1918 = while {
              stop <- w8273 stop-if-true
              n1919 = local read "Saving..."() -> (w8274:bool)
              n1920 = Not(x=w8274) -> (.not. x?=w8273:bool)
            }
          }
          frame #7 {
            n1921 = property on="Flip Green Filter" class="Bool (strict)"("Val(Sgnl)"=TRUE ("Value (Signaling)")) -> ()  [unwired: 2 in, 2 out]
            n1922 = property on="Green Laser ON/Interlacing" class="Bool (strict)"("Val(Sgnl)"=w8278) -> ()  [unwired: 2 in, 2 out]
            n1923 = property on="Green laser mode" class="RadioBtnsControl (strict)"("Val(Sgnl)"=w8277) -> ()  [unwired: 2 in, 2 out]
          }
          frame #8 {
            n1924 = property on="Green FB On/Off" class="Bool (strict)"("Val(Sgnl)"=w8279) -> ()  [unwired: 2 in, 2 out]
          }
        }
      }
      event "Stop All": Value Change {
        n1925 = event-data() -> ()  [unwired: 1 in, 5 out]
        n1926 = local read "Stop All"() -> (w8280:bool)
      }
    }
    n1927 = node-c288() -> ()  [unwired: 1 in, 1 out]
  }
  n1928 = timed-loop "Mouse control: trap position (AOM deflection), set confocal spot from image" {
    tunnel: [w8282] -> w169
    tunnel: w18 -> [w8281]
    timing: w67 -> [_]
    timing-out: [_] -> w66
    stop <- w8282 stop-if-true
    n1929 = node-c288() -> ()  [unwired: 2 out]
    n1930 = event shown="[1] \"Pane\": Mouse Move" {
      selector: _ -> [_ _]
      dyn-events: _ -> [_ _]
      timeout: _ -> [_ _]
      tunnel: w8281 -> [w8285 _]
      event Mouse Down {
        n1931 = event-data() -> ("Time"=w8287:u32, "Coords"=w8286:T8, "Button"=w8288:u16)  [unwired: 6 out]
        n1932 = case shown="1" w8288 {
          tunnel: w8287 -> [_ _ w8391]
          tunnel: w8286 -> [_ w8325 w8389]
          tunnel: w8285 -> [_ _ w8387]
          frame 0, Default {
          }
          frame 1 {
            n1933 = property on="APD 2" class="ImageControl"() -> ("Displayed Image Position"=w8295:cluster{"Left":i32, "Top":i32})  [unwired: 2 in, 2 out]
            n1934 = property on="APD 1" class="ImageControl"() -> ("Displayed Image Position"=w8324:cluster{"Left":i32, "Top":i32})  [unwired: 2 in, 2 out]
            n1935 = property on="Detection Laser X" class="ImageControl"() -> ("Displayed Image Position"=w8321:cluster{"Left":i32, "Top":i32})  [unwired: 2 in, 2 out]
            n1936 = property on="Detection Laser Y" class="ImageControl"() -> ("Displayed Image Position"=w8320:cluster{"Left":i32, "Top":i32})  [unwired: 2 in, 2 out]
            n1937 = property on="APD 2" class="ImageControl"() -> ("Displayed Image Size"=w8294:cluster{"Width":u32, "Height":u32})  [unwired: 2 in, 2 out]
            n1938 = property on="APD 1" class="ImageControl"() -> ("Displayed Image Size"=w8322:cluster{"Width":u32, "Height":u32})  [unwired: 2 in, 2 out]
            n1939 = property on="Detection Laser X" class="ImageControl"() -> ("Displayed Image Size"=w8323:cluster{"Width":u32, "Height":u32})  [unwired: 2 in, 2 out]
            n1940 = property on="Detection Laser Y" class="ImageControl"() -> ("Displayed Image Size"=w8319:cluster{"Width":u32, "Height":u32})  [unwired: 2 in, 2 out]
            n1941 = Unbundle By Name(w8294) -> ("Width"=w8291:u32, "Height"=w8290:u32)
            n1942 = Unbundle By Name(w8295) -> ("Left"=w8293:i32, "Top"=w8292:i32)
            n1943 = Unbundle By Name(w8322) -> ("Width"=w8316:u32, "Height"=w8315:u32)
            n1944 = Unbundle By Name(w8323) -> ("Width"=w8312:u32, "Height"=w8311:u32)
            n1945 = Unbundle By Name(w8319) -> ("Width"=w8308:u32, "Height"=w8307:u32)
            n1946 = Unbundle By Name(w8324) -> ("Left"=w8318:i32, "Top"=w8317:i32)
            n1947 = Unbundle By Name(w8321) -> ("Left"=w8314:i32, "Top"=w8313:i32)
            n1948 = Unbundle By Name(w8320) -> ("Left"=w8310:i32, "Top"=w8309:i32)
            n1949 = Bundle("Left"=w8293, "Top"=w8292, "Width"=w8291, "Height"=w8290) -> (w8289:T50)  [unwired: 1 in]
            n1950 = Bundle("Left"=w8318, "Top"=w8317, "Width"=w8316, "Height"=w8315) -> (w8306:T50)  [unwired: 1 in]
            n1951 = Bundle("Left"=w8314, "Top"=w8313, "Width"=w8312, "Height"=w8311) -> (w8305:T50)  [unwired: 1 in]
            n1952 = Bundle("Left"=w8310, "Top"=w8309, "Width"=w8308, "Height"=w8307) -> (w8304:T50)  [unwired: 1 in]
            n1953 = Build Cluster Array(w8289, w8306, w8305, w8304) -> (w8303:T51)
            n1954 = for {
              tunnel: w8325 -> [w8336]
              tunnel: w8303 -> [w8337] mode=indexing
              shift-right: [w8334] -> w8301
              shift-left: TRUE -> [w8335]
              shift-right: [w8333] -> w8299
              shift-left: _ -> [w8329]
              shift-right: [w8332] -> w8298
              shift-left: _ -> [w8328]
              shift-right: [w8331] -> w8297
              shift-left: _ -> [w8327]
              shift-right: [w8330] -> w8296
              shift-left: _ -> [w8326]
              n1955 = case shown="True" w8335 {
                selector: w8335 -> [w8342 _]
                tunnel: w8337 -> [_ w8351]
                tunnel: w8336 -> [_ w8349]
                tunnel: [w8342 w8347] -> w8334
                tunnel: [w8341 w8346] -> w8333
                tunnel: [w8340 w8345] -> w8332
                tunnel: [w8339 w8344] -> w8331
                tunnel: [w8338 w8343] -> w8330
                tunnel: w8329 -> [w8341 _]
                tunnel: w8328 -> [w8340 _]
                tunnel: w8327 -> [w8339 _]
                tunnel: w8326 -> [w8338 _]
                frame False {
                }
                frame True {
                  n1956 = Unbundle(w8351) -> (w8350:T50)
                  n1957 = call "isclickinwindow.vi"("Image Param"=w8350, "Point32"=w8349) -> ("4 Y"=w8343:i32, "3 Height"=w8344:i32, "2 X"=w8345:i32, "1 Width"=w8346:i32, "In image?"=w8348:bool)  [unwired: 1 in]
                  n1958 = Not(x=w8348) -> (.not. x?=w8347:bool)
                }
              }
            }
            n1959 = Not(x=w8301) -> (.not. x?=w8300:bool)
            n1960 = case shown="True" w8300 {
              tunnel: w8298 -> [_ w8364]
              tunnel: w8296 -> [_ w8363]
              tunnel: w8299 -> [_ w8362]
              tunnel: w8297 -> [_ w8361]
              frame False {
              }
              frame True {
                w8357 = FALSE ("Get Point")
                n1961 = local read "Scan lines (y)"() -> (w8366:u64)
                n1962 = local read "Actual MCL Inc (V)"() -> (w8358:dbl)
                n1963 = local read "Scan steps (MCL)"() -> (w8365:u64)
                n1964 = Divide "Y Pix/step"(x=w8361, y=w8366) -> (x/y=w8373:dbl)
                n1965 = Divide "Y V/pix"(x=w8358, y=w8373) -> (x/y=w8372:dbl)
                n1966 = Divide "Y half step offset"(x=w8358, y=2.0) -> (x/y=w8374:dbl)
                n1967 = Divide "X pix/step"(x=w8362, y=w8365) -> (x/y=w8371:dbl)
                n1968 = Negate(x=w8374) -> (-x=w8375:dbl)
                n1969 = local read "Initial Y"() -> (w8381:dbl)
                n1970 = Multiply(x=w8363, y=w8372) -> (x*y=w8382:dbl)
                n1971 = Divide "X half step offset"(x=w8358, y=2.0) -> (x/y=w8368:dbl)
                n1972 = Divide "X V/pix"(x=w8358, y=w8371) -> (x/y=w8370:dbl)
                n1973 = Multiply(x=w8358, y=w8365) -> (x*y=w8377:dbl)
                n1974 = Compound Arithmetic op=ADD(w8375, w8382, w8381) -> (w8359:dbl)
                "Pointer Y (V)" <- w8359
                n1975 = Multiply(x=w8370, y=w8364) -> (x*y=w8379:dbl)
                n1976 = Negate(x=w8368) -> (-x=w8367:dbl)
                n1977 = local read "Initial X"() -> (w8380:dbl)
                n1978 = Negate(x=w8379) -> (-x=w8378:dbl)
                n1979 = Compound Arithmetic op=ADD(w8367, w8377, w8380, w8378) -> (w8360:dbl)
                "Pointer X (V)" <- w8360
                n1980 = Or(x="Set X Only", y="Set Confocal Spot (X-Y)") -> (x .or. y?=w8353:bool)
                n1981 = Or(x="Set Confocal Spot (X-Y)", y="Set Y Only") -> (x .or. y?=w8352:bool)
                n1982 = case shown="True" w8353 {